vi "TCE_SaveConfiguration.vi"   [LabVIEW 2022 SP3] (continued)
"D, 220628_Psyringae_L_8days_c1_100fold_dil", "D, 220628_Psyringae_L_8days_c1_100fold_dil", "D, 220628_Psyringae_L_8days_c1_100fold_dil", "D, 220628_Psyringae_L_8days_c1_100fold_dil", "D, 220628_Psyringae_L_8days_c1_100fold_dil", "D, 220628_Psyringae_L_8days_c1_100fold_dil", "D, 220628_Psyringae_L_8days_c1_100fold_dil", "D, 220628_Psyringae_L_8days_c1_100fold_dil", "D, 220628_Psyringae_L_8days_c1_100fold_dil", "D, 220628_Psyringae_L_8days_c1_100fold_dil", "D, 220628_Psyringae_L_8days_c1_100fold_dil", "D, 220628_Psyringae_L_8days_c1_100fold_dil", "D, 220628_Psyringae_L_8days_c1_100fold_dil", "D, 220628_Psyringae_L_8days_c1_100fold_dil", "D, 220628_Psyringae_L_8days_c1_100fold_dil", "D, 220628_Psyringae_L_8days_c1_100fold_dil", "D, 220628_Psyringae_L_8days_c1_100fold_dil", "D, 220628_Psyringae_L_8days_c1_100fold_dil", "D, 220628_Psyringae_L_8days_c1_100fold_dil", "D, 220628_Psyringae_L_8days_c1_100fold_dil", "D, 220628_Psyringae_L_8days_c1_100fold_dil", "D, 220628_Psyringae_L_8days_c1_100fold_dil", "D, 220628_Psyringae_L_8days_c1_100fold_dil", "D, 220628_Psyringae_L_8days_c1_100fold_dil", "D, 220628_Psyringae_L_8days_c1_100fold_dil", "D, 220628_Psyringae_L_8days_c1_100fold_dil", "E, 220628_Psyringae_L_8days_c1_1000fold_dil", "E, 220628_Psyringae_L_8days_c1_1000fold_dil", "E, 220628_Psyringae_L_8days_c1_1000fold_dil", "E, 220628_Psyringae_L_8days_c1_1000fold_dil", "E, 220628_Psyringae_L_8days_c1_1000fold_dil", "E, 220628_Psyringae_L_8days_c1_1000fold_dil", "E, 220628_Psyringae_L_8days_c1_1000fold_dil", "E, 220628_Psyringae_L_8days_c1_1000fold_dil", "E, 220628_Psyringae_L_8days_c1_1000fold_dil", "E, 220628_Psyringae_L_8days_c1_1000fold_dil", "E, 220628_Psyringae_L_8days_c1_1000fold_dil", "E, 220628_Psyringae_L_8days_c1_1000fold_dil", "E, 220628_Psyringae_L_8days_c1_1000fold_dil", "E, 220628_Psyringae_L_8days_c1_1000fold_dil", "E, 220628_Psyringae_L_8days_c1_1000fold_dil", "E, 220628_Psyringae_L_8days_c1_1000fold_dil", "E, 220628_Psyringae_L_8days_c1_1000fold_dil", "E, 220628_Psyringae_L_8days_c1_1000fold_dil", "E, 220628_Psyringae_L_8days_c1_1000fold_dil", "E, 220628_Psyringae_L_8days_c1_1000fold_dil", "E, 220628_Psyringae_L_8days_c1_1000fold_dil", "E, 220628_Psyringae_L_8days_c1_1000fold_dil", "E, 220628_Psyringae_L_8days_c1_1000fold_dil", "E, 220628_Psyringae_L_8days_c1_1000fold_dil", "E, 220628_Psyringae_L_8days_c1_1000fold_dil", "E, 220628_Psyringae_L_8days_c1_1000fold_dil", "E, 220628_Psyringae_L_8days_c1_1000fold_dil", "E, 220628_Psyringae_L_8days_c1_1000fold_dil", "E, 220628_Psyringae_L_8days_c1_1000fold_dil", "E, 220628_Psyringae_L_8days_c1_1000fold_dil", "E, 220628_Psyringae_L_8days_c1_1000fold_dil", "E, 220628_Psyringae_L_8days_c1_1000fold_dil", "E, 220628_Psyringae_L_8days_c1_1000fold_dil", "E, 220628_Psyringae_L_8days_c1_1000fold_dil", "E, 220628_Psyringae_L_8days_c1_1000fold_dil", "E, 220628_Psyringae_L_8days_c1_1000fold_dil", "E, 220628_Psyringae_L_8days_c1_1000fold_dil", "E, 220628_Psyringae_L_8days_c1_1000fold_dil", "E, 220628_Psyringae_L_8days_c1_1000fold_dil", "E, 220628_Psyringae_L_8days_c1_1000fold_dil", "E, 220628_Psyringae_L_8days_c1_1000fold_dil", "E, 220628_Psyringae_L_8days_c1_1000fold_dil", "E, 220628_Psyringae_L_8days_c1_1000fold_dil", "E, 220628_Psyringae_L_8days_c1_1000fold_dil", "E, 220628_Psyringae_L_8days_c1_1000fold_dil", "E, 220628_Psyringae_L_8days_c1_1000fold_dil", "E, 220628_Psyringae_L_8days_c1_1000fold_dil", "E, 220628_Psyringae_L_8days_c1_1000fold_dil", "E, 220628_Psyringae_L_8days_c1_1000fold_dil", "E, 220628_Psyringae_L_8days_c1_1000fold_dil", "E, 220628_Psyringae_L_8days_c1_1000fold_dil", "E, 220628_Psyringae_L_8days_c1_1000fold_dil", "E, 220628_Psyringae_L_8days_c1_1000fold_dil", "E, 220628_Psyringae_L_8days_c1_1000fold_dil", "E, 220628_Psyringae_L_8days_c1_1000fold_dil", "E, 220628_Psyringae_L_8days_c1_1000fold_dil", "E, 220628_Psyringae_L_8days_c1_1000fold_dil", "E, 220628_Psyringae_L_8days_c1_1000fold_dil", "E, 220628_Psyringae_L_8days_c1_1000fold_dil", "E, 220628_Psyringae_L_8days_c1_1000fold_dil", "E, 220628_Psyringae_L_8days_c1_1000fold_dil", "E, 220628_Psyringae_L_8days_c1_1000fold_dil", "E, 220628_Psyringae_L_8days_c1_1000fold_dil", "E, 220628_Psyringae_L_8days_c1_1000fold_dil", "E, 220628_Psyringae_L_8days_c1_1000fold_dil", "E, 220628_Psyringae_L_8days_c1_1000fold_dil", "E, 220628_Psyringae_L_8days_c1_1000fold_dil", "E, 220628_Psyringae_L_8days_c1_1000fold_dil", "E, 220628_Psyringae_L_8days_c1_1000fold_dil", "E, 220628_Psyringae_L_8days_c1_1000fold_dil", "E, 220628_Psyringae_L_8days_c1_1000fold_dil", "E, 220628_Psyringae_L_8days_c1_1000fold_dil", "E, 220628_Psyringae_L_8days_c1_1000fold_dil", "E, 220628_Psyringae_L_8days_c1_1000fold_dil", "E, 220628_Psyringae_L_8days_c1_1000fold_dil", "E, 220628_Psyringae_L_8days_c1_1000fold_dil", "E, 220628_Psyringae_L_8days_c1_1000fold_dil", "E, 220628_Psyringae_L_8days_c1_1000fold_dil", "E, 220628_Psyringae_L_8days_c1_1000fold_dil", "E, 220628_Psyringae_L_8days_c1_1000fold_dil"], 7 "Offsets":dbl[](array[numeric])=[-0.90334019, -0.9161796, -0.80332393, -0.7834149, -0.82643058, -0.6685973, -0.74360948, -0.72258592, -0.70246108, -0.75416764, -0.73348982, -0.761681, -0.83858132, -0.76590043, -0.84169212, -0.79199164, -0.8463463, -0.76526398, -0.83821629, -0.91694116, -0.90690966, -0.68424699, -0.69370753, -0.71219233, -0.70905376, -0.67816346, -0.67457819, -0.62920248, -0.72726665, -0.69636261, -0.75405438, -0.67261546, -0.62911746, -0.69727554, -0.69403039, -0.74297488, -0.72961984, -0.73014797, -0.63921766, -0.68945531, -0.6339549, -0.64779226, -0.72921559, -0.75137744, -0.73587286, -0.72468758, -0.75455887, -0.6949301, -0.66419364, -0.78141906, -0.71708496, -0.74957072, -0.75440543, -0.79022752, -0.81582876, -0.85003708, -0.79718986, -0.70908029, -0.7948793, -0.82351793, -0.82099982, -0.90962242, -0.82940291, -0.82645972, -0.88457099, -0.90277854, -0.73435763, -0.89281041, -0.8731476, -0.90199506, -0.87104215, -0.93992167, -0.88914756, -0.90782778, -0.87556893, -0.89981662, -0.76902729, -0.83687477, -0.93247417, -0.86291953, -0.85195962, -0.81303577, -0.93169424, -0.88172655, -1.07267545, -0.97001875, -1.00105324, -1.00428899, -0.98393847, -1.03255942, -0.92122492, -1.07395808, -1.0128527, -1.05137684, -1.047103, -1.07584361, -1.07115095, -1.18445538, -1.07431948, -0.99711779, -1.05784667, -1.10645181, -1.12273395, -1.10840479, -1.15898328, -1.20715507, -1.14028285, -1.20342827, -1.24761428, -1.22032985, -1.27974244, -1.22850816, -1.26746488, -1.33153367, -1.14839422, -1.18404104, -1.23199741, -1.32498703, -1.26100096, -1.24243304, -1.2737479, -1.28610737, -1.30884853, -1.24839463, -1.16597388, -1.24925546, -1.16761645, -1.19659387, -1.21711949, -1.24061676, -1.26013109, -1.11073331, -1.22445389, -1.33253102, -1.20538906, -1.28740177, -1.38325577, -1.11760803, -1.28938927, -1.28976635, -1.36248042, -1.34015072, -1.31408804, -1.21046288, -1.25856053, -1.26922239, -1.15383794, -1.205826, -1.26086174, -1.23678076, -1.31317363, -1.37652076, -1.41586408, -1.20597583, -1.36710643, -1.34255233, -1.25131453, -1.2870645, -1.33174301, -1.40020549, -1.30694795, -1.2045447, -1.28020176, -1.42512079, -1.34800498, -1.42910301, -1.42657412, -1.40040383, -1.44534752, -1.31612798, -1.31328765, -1.2645929, -1.31730589, -1.44917086, -1.48042685, -1.48246777, -1.6069132, -1.49147634, -1.59657146, -1.49438681, -1.53218087, -1.61774453, -1.49481865, -1.46159514, -1.48785503, -1.59432746, -1.62819133, -1.71381539, -1.68348601, -1.7161616, -1.67665743, -1.68295333, -1.65154049, -1.52324358, -1.57369266, -1.5682697, -1.62700899, -1.71863545, -1.70241582, -1.75268931, -1.59710926, -1.66789895, -1.81990938, -1.72930759, -1.81298228, -1.74055081, -1.61731119, -1.73926896, -1.85620289, -1.73819272, -1.81750964, -1.82375387, -1.89273653, -1.88659901, -1.83943754, -1.79818326, -1.88636852, -1.69756045, -1.71421935, -1.87550076, -1.95622633, -1.83663434, -1.91914803, -1.91554095, -1.95163205, -1.89719334, -2.00565679, -1.88185899, -2.01510661, -2.02584106, -2.04327536, -2.00180772, -2.04674097, -1.96989144, -1.96809263, -2.05356691, -2.02755143, -2.04031214, -2.06345679, -2.05680446, -2.05412966, -2.07028399, -2.13129749, -2.19773722, -2.14798477, -2.02987559, -2.19712272, -2.12220486, -2.10896356, -2.17962118, -2.17513158, -2.16685523, -2.21700219, -2.10393398, -2.13717561, -2.2089672, -2.16493494, -2.18153417, -2.34229158, -2.16215572, -2.25785433, -2.22596349, -2.25187127, -2.35730309, -2.27379377, -2.32334743, -2.29175604, -2.20314771, -2.34439824, -2.38119664, -2.29790384, -2.40038917, -2.27058666, -2.40768479, -2.4473483, -2.60870625, -2.54751462, -2.53021285, -2.5877664, -2.41339714, -2.50834546, -2.61013394, -2.33705979, -2.54412908, -2.37872198, -2.32201169, -2.49044799, -2.48988715, -2.52837286, -2.4771429, -2.41691251, -2.41615598, -2.54943333, -2.44480101, -2.53825643, -2.40334417, -2.36938469, -2.37232876, -2.38218338, -2.4007207, -2.448537, -2.40978314, -2.50198391, -2.58420146, -2.48682817, -2.48172298, -2.45436571, -2.4967308, -2.43939981, -2.58457166, -2.43048312, -2.56066294, -2.45549519, -2.47804837, -2.42841964, -2.51133231, -2.44386246, -2.60310665, -2.67063121, -2.62883095, -2.64996527, -2.65067169, -2.71624159, -2.59601593, -2.74491664, -2.758366, -2.66158956, -2.63083217, -2.8731213, -2.8308766, -2.8027204, -2.7521968, -2.82272042, -2.8164733, -2.88768866, -2.90256896, -2.84367916, -2.9228607, -3.07481535, -2.88676048, -3.02662656, -2.95227409, -2.9718118, -2.96904895, -2.92507519, -2.90994016, -3.03592661, -2.86042929, -2.93424849, -2.86955675, -2.91288022, -2.92450324, -2.99792798, -3.05979151, -3.03700993, -2.93710315, -3.06990026, -2.98513574, -3.00533434, -2.97877259, -3.02315398, -3.08308014, -3.10903297, -3.15263997, -3.02982441, -3.26555892, -3.13993419, -3.41825506, -3.19378873, -3.23176941, -3.34563346, -3.29244211, -3.32094009, -3.41552083, -3.50898568, -3.28387452, -3.50556782, -3.49307458, -3.55551364, -3.45119325, -3.49144363, -3.35562487, -3.3305146, -3.49546844, -3.43299379, -3.43079581, -3.48817712, -3.52600011, -3.41451394, -3.45294882, -3.47961549, -3.50905251, -3.50087667, -3.62196941, -3.64036995, -3.66396678, -3.78242859, -3.8272262, -3.94477002, -3.94973945, -3.80467535, -3.85042978, -3.72641937, -3.77263417, -3.66180042, -3.91142471, -3.87559929, -3.81638351, -3.91497848, -3.9541892, -3.92320042, -3.99715778, -4.08213121, -4.02036058, -4.06936996, -3.94495614, -4.09507289, -4.03485348, -4.12562065, -4.23981777, -4.10507388, -4.21910866, -4.12512183, -4.28665132, -4.31376275, -4.18817295, -4.33383404, -4.36005697, -4.26141923, -4.18360141, -4.24917635, -4.35052763, -4.33966549, -4.38850899, -4.40321474, -4.49714659, -4.50771025, -4.51335601, -4.57639867, -4.42819556, -4.556029, -4.53683211, -4.47300718, -4.55151022, -4.67492457, -4.75698858, -4.63938981, -4.58238998, -4.66015878, -4.55188925, -4.6985391, -4.57481399], 9 "Offset Applied?":bool=TRUE) -> (14 "Save Array out":string[][](array[string]), 17 "Full Array":string[][](array[string]), 19 "Canceled":bool)   [LabVIEW 2022 SP3]
uses:
  DataCluster_TCAL.ctl
  <vilib>/vision/Image Controls.llb/IMAQ Image.ctl
  TCE_Config.ctl
panel:
  in  "Nm(T)":bool
  in  "SaveFrozen":bool=TRUE caption="Frozen Fraction"
  in  "SaveMelt":bool=TRUE caption="Melting Point"
  in  "SaveFreeze":bool=TRUE caption="Freezing Point"
  in  "SaveTemp":bool=TRUE caption="Temperatures"
  out "Data Array":string[][](array[string])
  in  "Cancel":bool
  in  "OK":bool
  # "Settings"
  # "File Preview"
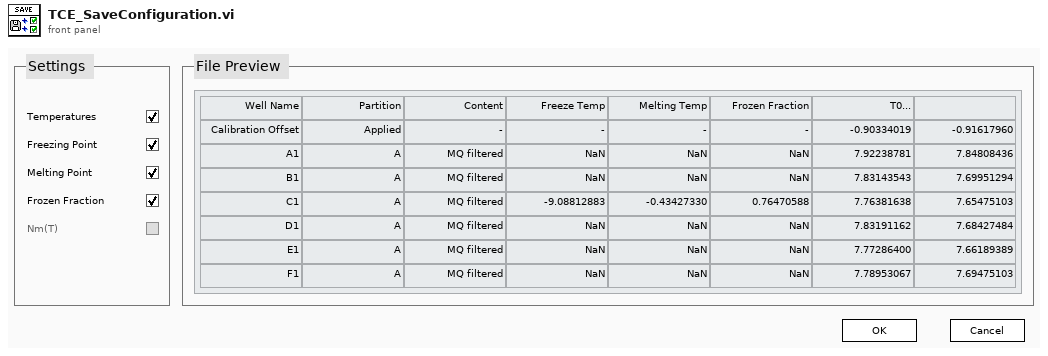
[diagram p1: front panel]
types:
  T1 = typedef "DataCluster_TCAL.ctl" = cluster{"Core":cluster{"Current VI Reference":refnum<vi>, "Close Panel on Exit?":bool}, "Image Out":T2, "State":i32, "Points":cluster{"Top Left":T3, "Top Right":T3, "Bottom Left":T3, "Bottom Right":T3, "x space 2":dbl, "y space 2":sgl, "x_space":sgl, "y_space":sgl, "Pixels":cluster{"X":i32, "Y":i32}[][], "Fixpoint":T3}, "img_array":T2[], "Temps":dbl[], "Temps_Array":dbl[][], "Scan Area":dbl, "Fixpoint Area":dbl, "Config":T4, "PCR Size":u16, "ImageCount":i32, "ShowGradient":bool}
  T2 = typedef "IMAQ Image.ctl" = refnum<image>
  T3 = typedef "IMAQ Point" = cluster{"X":sgl, "Y":sgl}
  T4 = typedef "TCE_Config.ctl" = cluster{"Freezing":cluster{"Cutoff":dbl, "EndIndex":i32}}
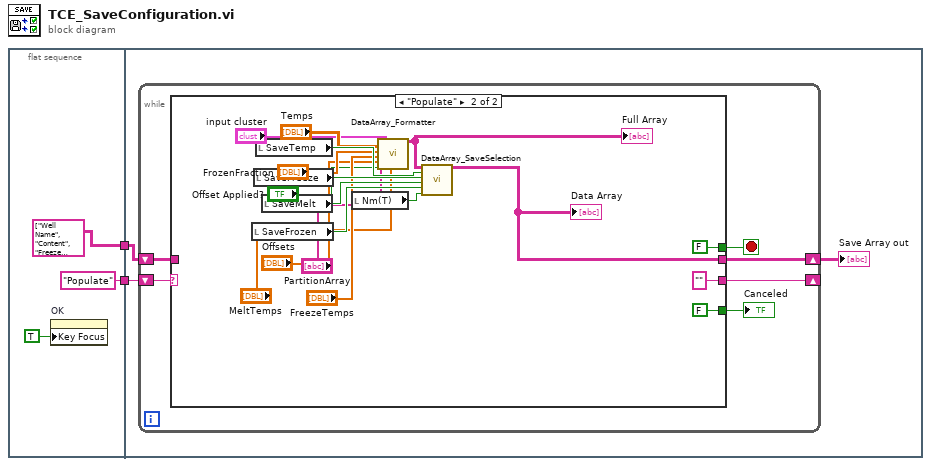
[diagram p0: block diagram]
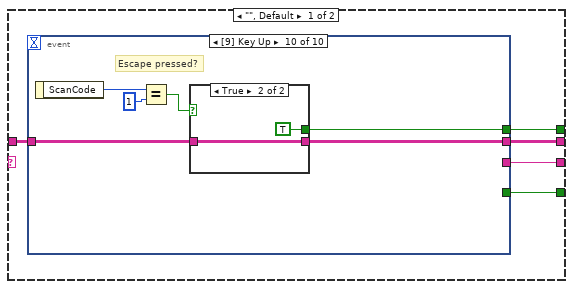
[diagram p2: hidden frame]
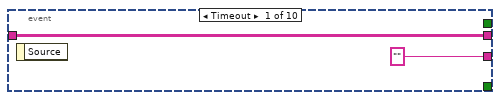
[diagram p3: hidden frame]
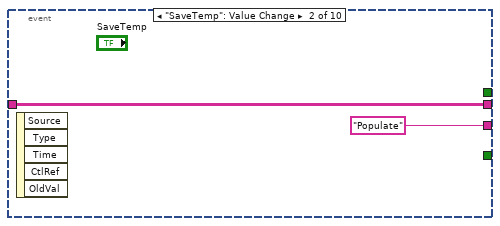
[diagram p4: hidden frame]
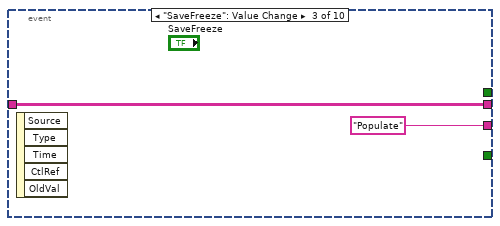
[diagram p5: hidden frame]
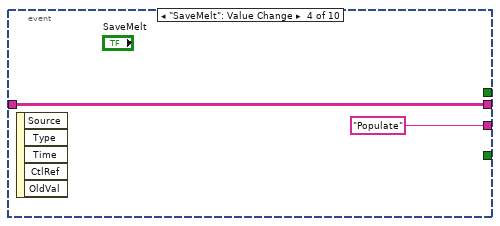
[diagram p6: hidden frame]
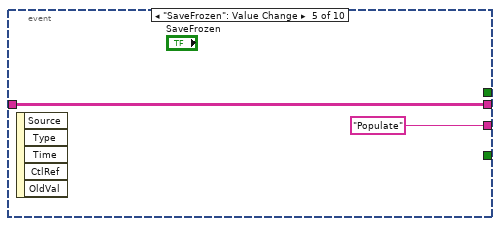
[diagram p7: hidden frame]
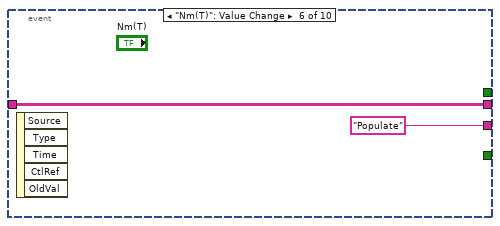
[diagram p8: hidden frame]
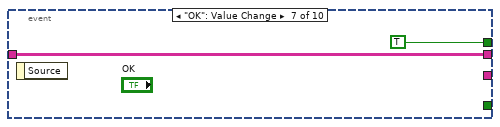
[diagram p9: hidden frame]
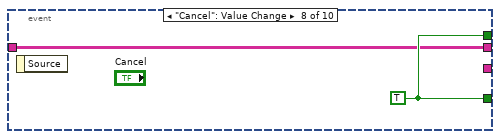
[diagram p10: hidden frame]
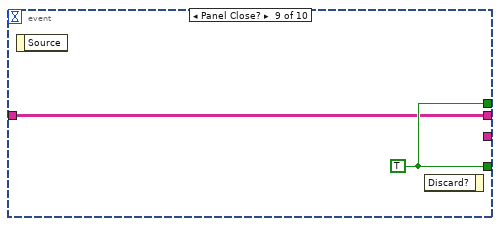
[diagram p11: hidden frame]
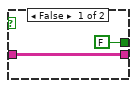
[diagram p12: hidden frame]
diagram:
  n1 = flat-sequence {
    tunnel: [string[][] [["Well Name", "Content", "Freeze Temp", "Melting Temp", "T0..."], ["Calibration Offset", "Not Applied", "", "", ""], ["A1", "", "", "", ""], ["B1", "", "", "", ""], ["C1", "", "", "", ""], ["D1", "", "", "", ""], ["E1", "", "", "", ""], ["F1", "", "", "", ""], ["G1", "", "", "", ""], ["H1", "", "", "", ""], ["I1", "", "", "", ""], ["J1", "", "", "", ""], ["K1", "", "", "", ""], ["L1", "", "", "", ""], ["M1", "", "", "", ""], ["N1", "", "", "", ""], ["O1", "", "", "", ""], ["P1", "", "", "", ""], ["A2", "", "", "", ""], ["B2", "", "", "", ""], ["C2", "", "", "", ""], ["D2", "", "", "", ""], ["E2", "", "", "", ""], ["F2", "", "", "", ""], ["G2", "", "", "", ""], ["H2", "", "", "", ""], ["I2", "", "", "", ""], ["J2", "", "", "", ""], ["K2", "", "", "", ""], ["L2", "", "", "", ""], ["M2", "", "", "", ""], ["N2", "", "", "", ""], ["O2", "", "", "", ""], ["P2", "", "", "", ""], ["A3", "", "", "", ""], ["B3", "", "", "", ""], ["C3", "", "", "", ""], ["D3", "", "", "", ""], ["E3", "", "", "", ""], ["F3", "", "", "", ""], ["G3", "", "", "", ""], ["H3", "", "", "", ""], ["I3", "", "", "", ""], ["J3", "", "", "", ""], ["K3", "", "", "", ""], ["L3", "", "", "", ""], ["M3", "", "", "", ""], ["N3", "", "", "", ""], ["O3", "", "", "", ""], ["P3", "", "", "", ""], ["A4", "", "", "", ""], ["B4", "", "", "", ""], ["C4", "", "", "", ""], ["D4", "", "", "", ""], ["E4", "", "", "", ""], ["F4", "", "", "", ""], ["G4", "", "", "", ""], ["H4", "", "", "", ""], ["I4", "", "", "", ""], ["J4", "", "", "", ""], ["K4", "", "", "", ""], ["L4", "", "", "", ""], ["M4", "", "", "", ""], ["N4", "", "", "", ""], ["O4", "", "", "", ""], ["P4", "", "", "", ""], ["A5", "", "", "", ""], ["B5", "", "", "", ""], ["C5", "", "", "", ""], ["D5", "", "", "", ""], ["E5", "", "", "", ""], ["F5", "", "", "", ""], ["G5", "", "", "", ""], ["H5", "", "", "", ""], ["I5", "", "", "", ""], ["J5", "", "", "", ""], ["K5", "", "", "", ""], ["L5", "", "", "", ""], ["M5", "", "", "", ""], ["N5", "", "", "", ""], ["O5", "", "", "", ""], ["P5", "", "", "", ""], ["A6", "", "", "", ""], ["B6", "", "", "", ""], ["C6", "", "", "", ""], ["D6", "", "", "", ""], ["E6", "", "", "", ""], ["F6", "", "", "", ""], ["G6", "", "", "", ""], ["H6", "", "", "", ""], ["I6", "", "", "", ""], ["J6", "", "", "", ""], ["K6", "", "", "", ""], ["L6", "", "", "", ""], ["M6", "", "", "", ""], ["N6", "", "", "", ""], ["O6", "", "", "", ""], ["P6", "", "", "", ""], ["A7", "", "", "", ""], ["B7", "", "", "", ""], ["C7", "", "", "", ""], ["D7", "", "", "", ""], ["E7", "", "", "", ""], ["F7", "", "", "", ""], ["G7", "", "", "", ""], ["H7", "", "", "", ""], ["I7", "", "", "", ""], ["J7", "", "", "", ""], ["K7", "", "", "", ""], ["L7", "", "", "", ""], ["M7", "", "", "", ""], ["N7", "", "", "", ""], ["O7", "", "", "", ""], ["P7", "", "", "", ""], ["A8", "", "", "", ""], ["B8", "", "", "", ""], ["C8", "", "", "", ""], ["D8", "", "", "", ""], ["E8", "", "", "", ""], ["F8", "", "", "", ""], ["G8", "", "", "", ""], ["H8", "", "", "", ""], ["I8", "", "", "", ""], ["J8", "", "", "", ""], ["K8", "", "", "", ""], ["L8", "", "", "", ""], ["M8", "", "", "", ""], ["N8", "", "", "", ""], ["O8", "", "", "", ""], ["P8", "", "", "", ""], ["A9", "", "", "", ""], ["B9", "", "", "", ""], ["C9", "", "", "", ""], ["D9", "", "", "", ""], ["E9", "", "", "", ""], ["F9", "", "", "", ""], ["G9", "", "", "", ""], ["H9", "", "", "", ""], ["I9", "", "", "", ""], ["J9", "", "", "", ""], ["K9", "", "", "", ""], ["L9", "", "", "", ""], ["M9", "", "", "", ""], ["N9", "", "", "", ""], ["O9", "", "", "", ""], ["P9", "", "", "", ""], ["A10", "", "", "", ""], ["B10", "", "", "", ""], ["C10", "", "", "", ""], ["D10", "", "", "", ""], ["E10", "", "", "", ""], ["F10", "", "", "", ""], ["G10", "", "", "", ""], ["H10", "", "", "", ""], ["I10", "", "", "", ""], ["J10", "", "", "", ""], ["K10", "", "", "", ""], ["L10", "", "", "", ""], ["M10", "", "", "", ""], ["N10", "", "", "", ""], ["O10", "", "", "", ""], ["P10", "", "", "", ""], ["A11", "", "", "", ""], ["B11", "", "", "", ""], ["C11", "", "", "", ""], ["D11", "", "", "", ""], ["E11", "", "", "", ""], ["F11", "", "", "", ""], ["G11", "", "", "", ""], ["H11", "", "", "", ""], ["I11", "", "", "", ""], ["J11", "", "", "", ""], ["K11", "", "", "", ""], ["L11", "", "", "", ""], ["M11", "", "", "", ""], ["N11", "", "", "", ""], ["O11", "", "", "", ""], ["P11", "", "", "", ""], ["A12", "", "", "", ""], ["B12", "", "", "", ""], ["C12", "", "", "", ""], ["D12", "", "", "", ""], ["E12", "", "", "", ""], ["F12", "", "", "", ""], ["G12", "", "", "", ""], ["H12", "", "", "", ""], ["I12", "", "", "", ""], ["J12", "", "", "", ""], ["K12", "", "", "", ""], ["L12", "", "", "", ""], ["M12", "", "", "", ""], ["N12", "", "", "", ""], ["O12", "", "", "", ""], ["P12", "", "", "", ""], ["A13", "", "", "", ""], ["B13", "", "", "", ""], ["C13", "", "", "", ""], ["D13", "", "", "", ""], ["E13", "", "", "", ""], ["F13", "", "", "", ""], ["G13", "", "", "", ""], ["H13", "", "", "", ""], ["I13", "", "", "", ""], ["J13", "", "", "", ""], ["K13", "", "", "", ""], ["L13", "", "", "", ""], ["M13", "", "", "", ""], ["N13", "", "", "", ""], ["O13", "", "", "", ""], ["P13", "", "", "", ""], ["A14", "", "", "", ""], ["B14", "", "", "", ""], ["C14", "", "", "", ""], ["D14", "", "", "", ""], ["E14", "", "", "", ""], ["F14", "", "", "", ""], ["G14", "", "", "", ""], ["H14", "", "", "", ""], ["I14", "", "", "", ""], ["J14", "", "", "", ""], ["K14", "", "", "", ""], ["L14", "", "", "", ""], ["M14", "", "", "", ""], ["N14", "", "", "", ""], ["O14", "", "", "", ""], ["P14", "", "", "", ""], ["A15", "", "", "", ""], ["B15", "", "", "", ""], ["C15", "", "", "", ""], ["D15", "", "", "", ""], ["E15", "", "", "", ""], ["F15", "", "", "", ""], ["G15", "", "", "", ""], ["H15", "", "", "", ""], ["I15", "", "", "", ""], ["J15", "", "", "", ""], ["K15", "", "", "", ""], ["L15", "", "", "", ""], ["M15", "", "", "", ""], ["N15", "", "", "", ""], ["O15", "", "", "", ""], ["P15", "", "", "", ""], ["A16", "", "", "", ""], ["B16", "", "", "", ""], ["C16", "", "", "", ""], ["D16", "", "", "", ""], ["E16", "", "", "", ""], ["F16", "", "", "", ""], ["G16", "", "", "", ""], ["H16", "", "", "", ""], ["I16", "", "", "", ""], ["J16", "", "", "", ""], ["K16", "", "", "", ""], ["L16", "", "", "", ""], ["M16", "", "", "", ""], ["N16", "", "", "", ""], ["O16", "", "", "", ""], ["P16", "", "", "", ""], ["A17", "", "", "", ""], ["B17", "", "", "", ""], ["C17", "", "", "", ""], ["D17", "", "", "", ""], ["E17", "", "", "", ""], ["F17", "", "", "", ""], ["G17", "", "", "", ""], ["H17", "", "", "", ""], ["I17", "", "", "", ""], ["J17", "", "", "", ""], ["K17", "", "", "", ""], ["L17", "", "", "", ""], ["M17", "", "", "", ""], ["N17", "", "", "", ""], ["O17", "", "", "", ""], ["P17", "", "", "", ""], ["A18", "", "", "", ""], ["B18", "", "", "", ""], ["C18", "", "", "", ""], ["D18", "", "", "", ""], ["E18", "", "", "", ""], ["F18", "", "", "", ""], ["G18", "", "", "", ""], ["H18", "", "", "", ""], ["I18", "", "", "", ""], ["J18", "", "", "", ""], ["K18", "", "", "", ""], ["L18", "", "", "", ""], ["M18", "", "", "", ""], ["N18", "", "", "", ""], ["O18", "", "", "", ""], ["P18", "", "", "", ""], ["A19", "", "", "", ""], ["B19", "", "", "", ""], ["C19", "", "", "", ""], ["D19", "", "", "", ""], ["E19", "", "", "", ""], ["F19", "", "", "", ""], ["G19", "", "", "", ""], ["H19", "", "", "", ""], ["I19", "", "", "", ""], ["J19", "", "", "", ""], ["K19", "", "", "", ""], ["L19", "", "", "", ""], ["M19", "", "", "", ""], ["N19", "", "", "", ""], ["O19", "", "", "", ""], ["P19", "", "", "", ""], ["A20", "", "", "", ""], ["B20", "", "", "", ""], ["C20", "", "", "", ""], ["D20", "", "", "", ""], ["E20", "", "", "", ""], ["F20", "", "", "", ""], ["G20", "", "", "", ""], ["H20", "", "", "", ""], ["I20", "", "", "", ""], ["J20", "", "", "", ""], ["K20", "", "", "", ""], ["L20", "", "", "", ""], ["M20", "", "", "", ""], ["N20", "", "", "", ""], ["O20", "", "", "", ""], ["P20", "", "", "", ""], ["A21", "", "", "", ""], ["B21", "", "", "", ""], ["C21", "", "", "", ""], ["D21", "", "", "", ""], ["E21", "", "", "", ""], ["F21", "", "", "", ""], ["G21", "", "", "", ""], ["H21", "", "", "", ""], ["I21", "", "", "", ""], ["J21", "", "", "", ""], ["K21", "", "", "", ""], ["L21", "", "", "", ""], ["M21", "", "", "", ""], ["N21", "", "", "", ""], ["O21", "", "", "", ""], ["P21", "", "", "", ""], ["A22", "", "", "", ""], ["B22", "", "", "", ""], ["C22", "", "", "", ""], ["D22", "", "", "", ""], ["E22", "", "", "", ""], ["F22", "", "", "", ""], ["G22", "", "", "", ""], ["H22", "", "", "", ""], ["I22", "", "", "", ""], ["J22", "", "", "", ""], ["K22", "", "", "", ""], ["L22", "", "", "", ""], ["M22", "", "", "", ""], ["N22", "", "", "", ""], ["O22", "", "", "", ""], ["P22", "", "", "", ""], ["A23", "", "", "", ""], ["B23", "", "", "", ""], ["C23", "", "", "", ""], ["D23", "", "", "", ""], ["E23", "", "", "", ""], ["F23", "", "", "", ""], ["G23", "", "", "", ""], ["H23", "", "", "", ""], ["I23", "", "", "", ""], ["J23", "", "", "", ""], ["K23", "", "", "", ""], ["L23", "", "", "", ""], ["M23", "", "", "", ""], ["N23", "", "", "", ""], ["O23", "", "", "", ""], ["P23", "", "", "", ""], ["A24", "", "", "", ""], ["B24", "", "", "", ""], ["C24", "", "", "", ""], ["D24", "", "", "", ""], ["E24", "", "", "", ""], ["F24", "", "", "", ""], ["G24", "", "", "", ""], ["H24", "", "", "", ""], ["I24", "", "", "", ""], ["J24", "", "", "", ""], ["K24", "", "", "", ""], ["L24", "", "", "", ""], ["M24", "", "", "", ""], ["N24", "", "", "", ""], ["O24", "", "", "", ""], ["P24", "", "", "", ""]] ("Data Array out")] -> w2
    tunnel: ["Populate"] -> w1
    tunnel: w2 -> [w8]
    tunnel: w1 -> [w7]
    frame #0 {
      n2 = property on="OK" class="Bool"("Key Focus"=TRUE) -> ()  [unwired: 2 in, 2 out]
    }
    frame #1 {
      n3 = while {
        shift-right: [w14] -> w6
        shift-left: w8 -> [w13]
        shift-right: [w9] -> _
        shift-left: w7 -> [w10]
        stop <- w12 stop-if-true
        n4 = case shown="\"Populate\"" w10 {
          tunnel: [w19 w48] -> w14
          tunnel: w13 -> [w18 _]
          tunnel: [w17 FALSE] -> w12
          tunnel: [w16 FALSE] -> w11
          tunnel: [w15 ""] -> w9
          frame "", Default {
            n5 = event shown="[9] Key Up" {
              selector: _ -> [_ _ _ _ _ _ _ _ _ _]
              dyn-events: _ -> [_ _ _ _ _ _ _ _ _ _]
              timeout: _ -> [_ _ _ _ _ _ _ _ _ _]
              tunnel: w18 -> [w20 w22 w24 w26 w28 w30 w33 w34 w36 w38]
              tunnel: [w20 w22 w24 w26 w28 w30 w33 w34 w36 w39] -> w19
              tunnel: [_ _ _ _ _ _ TRUE w35 w37 w43] -> w17
              tunnel: [_ _ _ _ _ _ _ w35 w37 _] -> w16
              tunnel: ["" "Populate" "Populate" "Populate" "Populate" "Populate" _ _ _ _] -> w15
              event Timeout {
                n6 = event-data() -> ()  [unwired: 1 in, 1 out]
              }
              event "SaveTemp": Value Change {
                n7 = event-data() -> ()  [unwired: 1 in, 5 out]
              }
              event "SaveFreeze": Value Change {
                n8 = event-data() -> ()  [unwired: 1 in, 5 out]
              }
              event "SaveMelt": Value Change {
                n9 = event-data() -> ()  [unwired: 1 in, 5 out]
              }
              event "SaveFrozen": Value Change {
                n10 = event-data() -> ()  [unwired: 1 in, 5 out]
              }
              event "Nm(T)": Value Change {
                n11 = event-data() -> ()  [unwired: 1 in, 5 out]
              }
              event "OK": Value Change {
                n12 = event-data() -> ()  [unwired: 1 in, 1 out]
              }
              event "Cancel": Value Change {
                w35 = TRUE
                n13 = event-data() -> ()  [unwired: 1 in, 1 out]
              }
              event Panel Close? {
                w37 = TRUE
                n14 = event-data() -> ()  [unwired: 1 in, 1 out]
                n15 = event-data() -> ()  [unwired: 2 in, 1 out]
              }
              event Key Up {
                # "Escape pressed?"
                n16 = event-data() -> ("ScanCode"=w42:i16)  [unwired: 1 in]
                n17 = Equal?(x=w42, y=i16 1) -> (x = y?=w40:bool)
                n18 = case shown="True" w40 {
                  tunnel: [FALSE TRUE] -> w43
                  tunnel: [w45 w46] -> w39
                  tunnel: w38 -> [w45 w46]
                  frame False {
                  }
                  frame True {
                  }
                }
              }
            }
          }
          frame "Populate" {
            n19 = local read "SaveFrozen"() -> (w59:bool)
            n20 = local read "SaveFreeze"() -> (w57:bool)
            n21 = local read "SaveTemp"() -> (w61:bool)
            n22 = local read "SaveMelt"() -> (w58:bool)
            n23 = local read "Nm(T)"() -> (w60:bool)
            n24 = call "DataArray_Formatter.vi"("PartitionArray"="PartitionArray", "Temps"="Temps", "FrozenFraction"="FrozenFraction", "FreezeTemps"="FreezeTemps", "Offsets"="Offsets", "Offset Applied?"="Offset Applied?", "input cluster"="input cluster", "MeltTemps"="MeltTemps") -> ("Data Array"=w62:string[][])  [unwired: 11 in]
            "Full Array" <- w62
            n25 = call "DataArray_SaveSelection.vi"("Data Array"=w62, "SaveTemp"=w61, "SaveFreeze"=w57, "SaveMelt"=w58, "SaveFrozen"=w59, "Nm(T)"=w60) -> ("Data Array out"=w48:string[][])  [unwired: 13 in]
            "Data Array" <- w48
          }
        }
        "Canceled" <- w11
      }
      "Save Array out" <- w6
    }
  }
